vi "Dresden R2R Sputter 03.02.2018 IY24.vi"() -> ()   [LabVIEW 2009] (continued)
                                frame #1 {
                                }
                                }
                                }
                                }
                                }
                                frame #1 {
                                n30610 = stacked-sequence {
                                frame #0 {
                                n30611 = local write "Transfer_ch3_2"(TRUE ("Transfer_ch3_2")) -> ()
                                n30612 = Wait (ms)(milliseconds to wait=u32 100) -> ()  [unwired: 1 out]
                                }
                                frame #1 {
                                n30613 = while {
                                stop <- w35437 stop-if-true
                                n30614 = Wait Until Next ms Multiple(millisecond multiple=u32 300) -> ()  [unwired: 1 out]
                                n30615 = local read "Transfer_ch3_2"() -> (w35438:bool)
                                n30616 = local read "Semi"() -> (w35440:bool)
                                n30617 = Not(x=w35438) -> (.not. x?=w35439:bool)
                                n30618 = Or(x=w35439, y=w35440) -> (x .or. y?=w35437:bool)
                                }
                                }
                                }
                                }
                                frame #2 {
                                n30619 = local read "Single_Ch2_Interlock"() -> (w35441:dbl)
                                n30620 = local read "Ch2_pressure"() -> (w35445:dbl)
                                n30621 = local read "started_up_ch2"() -> (w35443:bool)
                                n30622 = In Range and Coerce(upper limit=w35441, x=w35445, lower limit=1e-08) -> (In Range?=w35446:bool)  [unwired: 1 out]
                                n30623 = And(x=w35446, y=w35443) -> (x .and. y?=w35442:bool)
                                n30624 = case shown="True" w35442 {
                                frame #0 {
                                }
                                frame #1 {
                                n30625 = local read "Semi"() -> (w35447:bool)
                                n30626 = case shown="False" w35447 {
                                frame #0 {
                                n30627 = stacked-sequence {
                                frame #0 {
                                # "WATER FLOW CONTROL OPEN"
                                n30628 = stacked-sequence {
                                frame #0 {
                                n30629 = local read "Semi"() -> (w35448:bool)
                                n30630 = case shown="False" w35448 {
                                frame #0 {
                                n30631 = while {
                                i -> [w35454]
                                stop <- w35449 stop-if-true
                                n30632 = Greater?(x=w35454, y=100) -> (0:w35453:bool)
                                n30633 = case shown="True" w35453 {
                                frame #0 {
                                }
                                frame #1 {
                                n30634 = local write "Semi"(TRUE ("Semi")) -> ()
                                n30635 = local write "Error Message"("Coating Process  \nwas cancelled.\nPlease check water \nflow connection." ("Error Message")) -> ()
                                }
                                }
                                n30636 = local read "Ch4_WFS_di"() -> (w35452:bool)
                                n30637 = case shown="True" w35452 {
                                tunnel: [TRUE FALSE] -> w35451
                                frame #0 {
                                }
                                frame #1 {
                                n30638 = local write "Ch4_WFC_do"(FALSE ("Ch1_WFC_do")) -> ()
                                n30639 = Wait Until Next ms Multiple(millisecond multiple=u32 200) -> ()  [unwired: 1 out]
                                }
                                }
                                n30640 = local read "Semi"() -> (w35450:bool)
                                n30641 = Or(x=w35451, y=w35450) -> (x .or. y?=w35449:bool)
                                }
                                }
                                frame #1 {
                                }
                                }
                                }
                                frame #1 {
                                n30642 = local read "Semi"() -> (w35462:bool)
                                n30643 = case shown="False" w35462 {
                                frame #0 {
                                n30644 = while {
                                i -> [w35468]
                                stop <- w35463 stop-if-true
                                n30645 = Greater?(x=w35468, y=100) -> (0:w35467:bool)
                                n30646 = case shown="True" w35467 {
                                frame #0 {
                                }
                                frame #1 {
                                n30647 = local write "Semi"(TRUE ("Semi")) -> ()
                                n30648 = local write "Error Message"("Coating Process  \nwas cancelled.\nPlease check water \nflow connection." ("Error Message")) -> ()
                                }
                                }
                                n30649 = local read "Ch3_WFS_di"() -> (w35466:bool)
                                n30650 = case shown="True" w35466 {
                                tunnel: [TRUE FALSE] -> w35465
                                frame #0 {
                                }
                                frame #1 {
                                n30651 = local write "Ch3_WFC_do"(FALSE ("Ch1_WFC_do")) -> ()
                                n30652 = Wait Until Next ms Multiple(millisecond multiple=u32 200) -> ()  [unwired: 1 out]
                                }
                                }
                                n30653 = local read "Semi"() -> (w35464:bool)
                                n30654 = Or(x=w35465, y=w35464) -> (x .or. y?=w35463:bool)
                                }
                                }
                                frame #1 {
                                }
                                }
                                }
                                frame #2 {
                                n30655 = local read "Semi"() -> (w35476:bool)
                                n30656 = case shown="False" w35476 {
                                frame #0 {
                                n30657 = while {
                                i -> [w35482]
                                stop <- w35477 stop-if-true
                                n30658 = Greater?(x=w35482, y=100) -> (0:w35481:bool)
                                n30659 = case shown="True" w35481 {
                                frame #0 {
                                }
                                frame #1 {
                                n30660 = local write "Semi"(TRUE ("Semi")) -> ()
                                n30661 = local write "Error Message"("Coating Process  \nwas cancelled.\nPlease check water \nflow connection." ("Error Message")) -> ()
                                }
                                }
                                n30662 = local read "Ch1_WFS_di"() -> (w35480:bool)
                                n30663 = case shown="True" w35480 {
                                tunnel: [TRUE FALSE] -> w35479
                                frame #0 {
                                }
                                frame #1 {
                                n30664 = local write "Ch1_WFC_do"(FALSE ("Ch1_WFC_do")) -> ()
                                n30665 = Wait Until Next ms Multiple(millisecond multiple=u32 200) -> ()  [unwired: 1 out]
                                }
                                }
                                n30666 = local read "Semi"() -> (w35478:bool)
                                n30667 = Or(x=w35479, y=w35478) -> (x .or. y?=w35477:bool)
                                }
                                }
                                frame #1 {
                                }
                                }
                                }
                                frame #3 {
                                n30668 = local read "Semi"() -> (w35490:bool)
                                n30669 = case shown="False" w35490 {
                                frame #0 {
                                n30670 = while {
                                i -> [w35496]
                                stop <- w35491 stop-if-true
                                n30671 = Greater?(x=w35496, y=100) -> (0:w35495:bool)
                                n30672 = case shown="True" w35495 {
                                frame #0 {
                                }
                                frame #1 {
                                n30673 = local write "Semi"(TRUE ("Semi")) -> ()
                                n30674 = local write "Error Message"("Coating Process  \nwas cancelled.\nPlease check water \nflow connection." ("Error Message")) -> ()
                                }
                                }
                                n30675 = local read "Ch2_WFS_di"() -> (w35494:bool)
                                n30676 = case shown="False" w35494 {
                                tunnel: [FALSE TRUE] -> w35493
                                frame #0 {
                                n30677 = local write "Ch2_WFC_do"(TRUE ("Ch1_WFC_do")) -> ()
                                n30678 = Wait Until Next ms Multiple(millisecond multiple=u32 200) -> ()  [unwired: 1 out]
                                }
                                frame #1 {
                                }
                                }
                                n30679 = local read "Semi"() -> (w35492:bool)
                                n30680 = Or(x=w35493, y=w35492) -> (x .or. y?=w35491:bool)
                                }
                                }
                                frame #1 {
                                }
                                }
                                }
                                frame #4 {
                                n30681 = local read "Semi"() -> (w35504:bool)
                                n30682 = case shown="False" w35504 {
                                frame #0 {
                                n30683 = local write "SDC1 2"(TRUE ("SDC1 2")) -> ()
                                n30684 = Wait (ms)(milliseconds to wait=u32 1000) -> ()  [unwired: 1 out]
                                }
                                frame #1 {
                                }
                                }
                                }
                                }
                                }
                                frame #1 {
                                # "BG-BV open"
                                n30685 = stacked-sequence {
                                frame #0 {
                                n30686 = local read "Semi"() -> (w35507:bool)
                                n30687 = case shown="False" w35507 {
                                frame #0 {
                                n30688 = while {
                                i -> [w35513]
                                stop <- w35508 stop-if-true
                                n30689 = Greater?(x=w35513, y=50) -> (0:w35512:bool)
                                n30690 = case shown="True" w35512 {
                                frame #0 {
                                }
                                frame #1 {
                                n30691 = local write "Semi"(TRUE ("Semi")) -> ()
                                n30692 = local write "Error Message"("Coating Process  \nwas cancelled.\nPlease check \nBG-BV connection." ("Error Message")) -> ()
                                }
                                }
                                n30693 = local read "Ch2_Bg_bv_di"() -> (w35511:bool)
                                n30694 = case shown="False" w35511 {
                                tunnel: [FALSE TRUE] -> w35510
                                frame #0 {
                                n30695 = local write "Ch2_Bg_bv_do"(TRUE ("Ch1_WFC_do")) -> ()
                                n30696 = Wait Until Next ms Multiple(millisecond multiple=u32 200) -> ()  [unwired: 1 out]
                                }
                                frame #1 {
                                }
                                }
                                n30697 = local read "Semi"() -> (w35509:bool)
                                n30698 = Or(x=w35510, y=w35509) -> (x .or. y?=w35508:bool)
                                }
                                }
                                frame #1 {
                                }
                                }
                                }
                                frame #1 {
                                n30699 = local read "Semi"() -> (w35521:bool)
                                n30700 = case shown="False" w35521 {
                                frame #0 {
                                n30701 = Wait (ms)(milliseconds to wait=u32 1000) -> ()  [unwired: 1 out]
                                n30702 = local write "SDC1 4"(TRUE ("SDC1 4")) -> ()
                                }
                                frame #1 {
                                }
                                }
                                }
                                }
                                }
                                frame #2 {
                                # "Baratron set zero"
                                n30703 = stacked-sequence {
                                frame #0 {
                                n30704 = local write "Pc_bv2_auto_baratron_set_zero"(TRUE ("Pc_bv2_auto_baratron_set_zero")) -> ()
                                }
                                frame #1 {
                                n30705 = while {
                                i -> [w35528]
                                stop <- w35525 stop-if-true
                                n30706 = Greater?(x=w35528, y=50 ("Baratron set zero time")) -> (0:w35527:bool)
                                n30707 = case shown="True" w35527 {
                                frame #0 {
                                }
                                frame #1 {
                                n30708 = local write "Semi"(TRUE ("Semi")) -> ()
                                n30709 = local write "Error Message"("" ("Error Message")) -> ()
                                }
                                }
                                n30710 = local read "Pressure 2"() -> (w35533:i32)
                                n30711 = Less?(x=w35533, y=0.1 ("Pressure Check for baratron set zero")) -> (x < y?=w35531:bool)
                                n30712 = case shown="False" w35531 {
                                tunnel: [FALSE TRUE] -> w35530
                                frame #0 {
                                n30713 = Wait Until Next ms Multiple(millisecond multiple=u32 200) -> ()  [unwired: 1 out]
                                }
                                frame #1 {
                                }
                                }
                                n30714 = local read "Semi"() -> (w35529:bool)
                                n30715 = Or(x=w35530, y=w35529) -> (x .or. y?=w35525:bool)
                                }
                                }
                                frame #2 {
                                n30716 = local read "Semi"() -> (w35539:bool)
                                n30717 = case shown="False" w35539 {
                                frame #0 {
                                n30718 = local write "SDC1 2b"(TRUE ("SDC1 2b")) -> ()
                                n30719 = Wait (ms)(milliseconds to wait=u32 1000) -> ()  [unwired: 1 out]
                                }
                                frame #1 {
                                }
                                }
                                }
                                }
                                }
                                frame #3 {
                                # "CC CLOSE"
                                n30720 = stacked-sequence {
                                frame #0 {
                                n30721 = local read "Semi"() -> (w35542:bool)
                                n30722 = case shown="False" w35542 {
                                frame #0 {
                                n30723 = while {
                                i -> [w35548]
                                stop <- w35543 stop-if-true
                                n30724 = Greater?(x=w35548, y=50) -> (0:w35547:bool)
                                n30725 = case shown="True" w35547 {
                                frame #0 {
                                }
                                frame #1 {
                                n30726 = local write "Semi"(TRUE ("Semi")) -> ()
                                n30727 = local write "Error Message"("Coating Process  \nwas cancelled.\nPlease check \nBG-BV connection." ("Error Message")) -> ()
                                }
                                }
                                n30728 = local read "Ch2_Cc_on_off_di"() -> (w35546:bool)
                                n30729 = case shown="True" w35546 {
                                tunnel: [TRUE FALSE] -> w35545
                                frame #0 {
                                }
                                frame #1 {
                                n30730 = local write "Ch2_Cc_on_off_do"(FALSE ("Ch1_WFC_do")) -> ()
                                n30731 = Wait Until Next ms Multiple(millisecond multiple=u32 200) -> ()  [unwired: 1 out]
                                }
                                }
                                n30732 = local read "Semi"() -> (w35544:bool)
                                n30733 = Or(x=w35545, y=w35544) -> (x .or. y?=w35543:bool)
                                }
                                }
                                frame #1 {
                                }
                                }
                                }
                                frame #1 {
                                n30734 = local read "Semi"() -> (w35556:bool)
                                n30735 = case shown="False" w35556 {
                                frame #0 {
                                n30736 = local write "SDC1 3"(TRUE ("SDC1 3")) -> ()
                                n30737 = Wait (ms)(milliseconds to wait=u32 1000) -> ()  [unwired: 1 out]
                                }
                                frame #1 {
                                }
                                }
                                }
                                }
                                }
                                frame #4 {
                                # "PC-BV CLOSE"
                                n30738 = stacked-sequence {
                                frame #0 {
                                n30739 = local read "Semi"() -> (w35559:bool)
                                n30740 = case shown="False" w35559 {
                                frame #0 {
                                n30741 = stacked-sequence {
                                frame #0 {
                                n30742 = local read "Semi"() -> (w35560:bool)
                                n30743 = case shown="False" w35560 {
                                frame #0 {
                                n30744 = local write "Pc_bv2_auto_close"(TRUE ("Tp1_auto_start")) -> ()
                                }
                                frame #1 {
                                }
                                }
                                }
                                frame #1 {
                                n30745 = local read "Semi"() -> (w35562:bool)
                                n30746 = case shown="False" w35562 {
                                frame #0 {
                                n30747 = Wait (ms)(milliseconds to wait=u32 1000) -> ()  [unwired: 1 out]
                                }
                                frame #1 {
                                }
                                }
                                }
                                frame #2 {
                                n30748 = local read "Semi"() -> (w35564:bool)
                                n30749 = case shown="False" w35564 {
                                frame #0 {
                                n30750 = while {
                                i -> [w35570]
                                stop <- w35566 stop-if-true
                                n30751 = local read "Pc_bv_closed_ch2"() -> (w35568:bool)
                                n30752 = Greater?(x=w35570, y=120) -> (0:w35569:bool)
                                n30753 = local read "Semi"() -> (w35567:bool)
                                n30754 = Compound Arithmetic op=OR(w35567, w35568, w35569) -> (w35566:bool)
                                n30755 = Wait (ms)(milliseconds to wait=u32 500) -> ()  [unwired: 1 out]
                                }
                                }
                                frame #1 {
                                }
                                }
                                }
                                frame #3 {
                                n30756 = local read "Semi"() -> (w35572:bool)
                                n30757 = case shown="False" w35572 {
                                frame #0 {
                                n30758 = local read "Pc_bv_closed_ch2"() -> (w35573:bool)
                                n30759 = case shown="False" w35573 {
                                frame #0 {
                                n30760 = local write "Pc_bv2_auto_close"(TRUE ("Pc_bv1_auto_open")) -> ()
                                }
                                frame #1 {
                                }
                                }
                                }
                                frame #1 {
                                }
                                }
                                }
                                frame #4 {
                                n30761 = local read "Semi"() -> (w35575:bool)
                                n30762 = case shown="False" w35575 {
                                frame #0 {
                                n30763 = local read "Pc_bv_closed_ch2"() -> (w35576:bool)
                                n30764 = case shown="False" w35576 {
                                frame #0 {
                                n30765 = Wait (ms)(milliseconds to wait=u32 1000) -> ()  [unwired: 1 out]
                                }
                                frame #1 {
                                }
                                }
                                }
                                frame #1 {
                                }
                                }
                                }
                                frame #5 {
                                n30766 = local read "Semi"() -> (w35578:bool)
                                n30767 = case shown="False" w35578 {
                                frame #0 {
                                n30768 = while {
                                i -> [w35584]
                                stop <- w35580 stop-if-true
                                n30769 = local read "Pc_bv_closed_ch2"() -> (w35582:bool)
                                n30770 = Greater?(x=w35584, y=120) -> (0:w35583:bool)
                                n30771 = local read "Semi"() -> (w35581:bool)
                                n30772 = Compound Arithmetic op=OR(w35581, w35582, w35583) -> (w35580:bool)
                                n30773 = Wait (ms)(milliseconds to wait=u32 500) -> ()  [unwired: 1 out]
                                }
                                }
                                frame #1 {
                                }
                                }
                                }
                                frame #6 {
                                n30774 = local read "Semi"() -> (w35586:bool)
                                n30775 = case shown="False" w35586 {
                                frame #0 {
                                n30776 = local read "Pc_bv_closed_ch2"() -> (w35587:bool)
                                n30777 = case shown="False" w35587 {
                                frame #0 {
                                n30778 = local write "Error Message"("Start up process  cancelled\nbecause  PC-BV not closed.\nPlease check PC-BV1 connections." ("Error Message")) -> ()
                                n30779 = Wait (ms)(milliseconds to wait=u32 1000) -> ()  [unwired: 1 out]
                                }
                                frame #1 {
                                }
                                }
                                }
                                frame #1 {
                                }
                                }
                                }
                                }
                                }
                                frame #1 {
                                }
                                }
                                }
                                frame #1 {
                                n30780 = local read "Semi"() -> (w35590:bool)
                                n30781 = case shown="False" w35590 {
                                frame #0 {
                                n30782 = local write "SDC1 5"(TRUE ("SDC1 5")) -> ()
                                n30783 = Wait (ms)(milliseconds to wait=u32 1000) -> ()  [unwired: 1 out]
                                }
                                frame #1 {
                                }
                                }
                                }
                                }
                                }
                                frame #5 {
                                # "SOV-AR OPEN"
                                n30784 = stacked-sequence {
                                frame #0 {
                                n30785 = local read "Semi"() -> (w35593:bool)
                                n30786 = case shown="False" w35593 {
                                frame #0 {
                                n30787 = while {
                                i -> [w35599]
                                stop <- w35594 stop-if-true
                                n30788 = Greater?(x=w35599, y=50) -> (0:w35598:bool)
                                n30789 = case shown="True" w35598 {
                                frame #0 {
                                }
                                frame #1 {
                                n30790 = local write "Semi"(TRUE ("Semi")) -> ()
                                n30791 = local write "Error Message"("Coating Process  \nwas cancelled.\nPlease check \nSOV-Ar connection." ("Error Message")) -> ()
                                }
                                }
                                n30792 = local read "Ch2_Sov_Ar_di"() -> (w35597:bool)
                                n30793 = case shown="False" w35597 {
                                tunnel: [FALSE TRUE] -> w35596
                                frame #0 {
                                n30794 = local write "Ch2_Sov_Ar_do"(TRUE ("Ch1_WFC_do")) -> ()
                                n30795 = Wait Until Next ms Multiple(millisecond multiple=u32 200) -> ()  [unwired: 1 out]
                                }
                                frame #1 {
                                }
                                }
                                n30796 = local read "Semi"() -> (w35595:bool)
                                n30797 = Or(x=w35596, y=w35595) -> (x .or. y?=w35594:bool)
                                }
                                }
                                frame #1 {
                                }
                                }
                                }
                                frame #1 {
                                n30798 = local read "Semi"() -> (w35607:bool)
                                n30799 = case shown="False" w35607 {
                                frame #0 {
                                n30800 = while {
                                i -> [w35612]
                                stop <- w35610 stop-if-true
                                n30801 = Greater?(x=w35612, y=5) -> (0:w35608:bool)
                                n30802 = Wait Until Next ms Multiple(millisecond multiple=u32 1000) -> ()  [unwired: 1 out]
                                n30803 = local read "Semi"() -> (w35611:bool)
                                n30804 = Or(x=w35608, y=w35611) -> (x .or. y?=w35610:bool)
                                }
                                }
                                frame #1 {
                                }
                                }
                                }
                                frame #2 {
                                n30805 = local read "Semi"() -> (w35614:bool)
                                n30806 = case shown="False" w35614 {
                                frame #0 {
                                n30807 = local write "SDC1 6"(TRUE ("SDC1 6")) -> ()
                                n30808 = Wait (ms)(milliseconds to wait=u32 1000) -> ()  [unwired: 1 out]
                                }
                                frame #1 {
                                }
                                }
                                }
                                }
                                }
                                frame #6 {
                                # "CHECK CHAMBER PRESSURE"
                                n30809 = stacked-sequence {
                                frame #0 {
                                n30810 = local read "Semi"() -> (w35617:bool)
                                n30811 = case shown="False" w35617 {
                                frame #0 {
                                n30812 = while {
                                i -> [w35625]
                                stop <- w35619 stop-if-true
                                n30813 = Greater?(x=w35625, y=300) -> (0:w35624:bool)
                                n30814 = case shown="True" w35624 {
                                frame #0 {
                                }
                                frame #1 {
                                n30815 = local write "Semi"(TRUE ("Semi")) -> ()
                                n30816 = local write "Error Message"("Coating Process cancelled.\nPlease check chamber \nconnections." ("Error Message")) -> ()
                                }
                                }
                                n30817 = local read "Ch_pg_press_ch2_gui 2"() -> (w35618:dbl)
                                n30818 = Greater Or Equal?(x=w35618, y=0.9 ("CHAMBER PRESSURE 4")) -> (x >= y?=w35622:bool)
                                n30819 = case shown="True" w35622 {
                                tunnel: [TRUE FALSE] -> w35621
                                frame #0 {
                                }
                                frame #1 {
                                n30820 = Wait Until Next ms Multiple(millisecond multiple=u32 200) -> ()  [unwired: 1 out]
                                }
                                }
                                n30821 = local read "Semi"() -> (w35620:bool)
                                n30822 = Or(x=w35621, y=w35620) -> (x .or. y?=w35619:bool)
                                }
                                }
                                frame #1 {
                                }
                                }
                                }
                                frame #1 {
                                n30823 = local read "Semi"() -> (w35632:bool)
                                n30824 = case shown="False" w35632 {
                                frame #0 {
                                n30825 = Wait (ms)(milliseconds to wait=u32 1000) -> ()  [unwired: 1 out]
                                n30826 = local write "SDC1 8"(TRUE ("SDC1 8")) -> ()
                                }
                                frame #1 {
                                }
                                }
                                }
                                }
                                }
                                frame #7 {
                                # "PC-BV OPEN"
                                n30827 = stacked-sequence {
                                frame #0 {
                                n30828 = local read "Semi"() -> (w35635:bool)
                                n30829 = case shown="False" w35635 {
                                frame #0 {
                                n30830 = stacked-sequence {
                                frame #0 {
                                n30831 = local read "Semi"() -> (w35636:bool)
                                n30832 = case shown="False" w35636 {
                                frame #0 {
                                n30833 = local write "Pc_bv2_auto_open"(TRUE ("Tp1_auto_start")) -> ()
                                }
                                frame #1 {
                                }
                                }
                                }
                                frame #1 {
                                n30834 = local read "Semi"() -> (w35638:bool)
                                n30835 = case shown="False" w35638 {
                                frame #0 {
                                n30836 = Wait (ms)(milliseconds to wait=u32 1000) -> ()  [unwired: 1 out]
                                }
                                frame #1 {
                                }
                                }
                                }
                                frame #2 {
                                n30837 = local read "Semi"() -> (w35640:bool)
                                n30838 = case shown="False" w35640 {
                                frame #0 {
                                n30839 = while {
                                i -> [w35646]
                                stop <- w35642 stop-if-true
                                n30840 = local read "Pc_bv_opened_ch2"() -> (w35644:bool)
                                n30841 = Greater?(x=w35646, y=120) -> (0:w35645:bool)
                                n30842 = local read "Semi"() -> (w35643:bool)
                                n30843 = Compound Arithmetic op=OR(w35643, w35644, w35645) -> (w35642:bool)
                                n30844 = Wait (ms)(milliseconds to wait=u32 500) -> ()  [unwired: 1 out]
                                }
                                }
                                frame #1 {
                                }
                                }
                                }
                                frame #3 {
                                n30845 = local read "Semi"() -> (w35648:bool)
                                n30846 = case shown="False" w35648 {
                                frame #0 {
                                n30847 = local read "Pc_bv_opened_ch2"() -> (w35649:bool)
                                n30848 = case shown="False" w35649 {
                                frame #0 {
                                n30849 = local write "Pc_bv2_auto_open"(TRUE ("Pc_bv1_auto_open")) -> ()
                                }
                                frame #1 {
                                }
                                }
                                }
                                frame #1 {
                                }
                                }
                                }
                                frame #4 {
                                n30850 = local read "Semi"() -> (w35651:bool)
                                n30851 = case shown="False" w35651 {
                                frame #0 {
                                n30852 = local read "Pc_bv_opened_ch2"() -> (w35652:bool)
                                n30853 = case shown="False" w35652 {
                                frame #0 {
                                n30854 = Wait (ms)(milliseconds to wait=u32 1000) -> ()  [unwired: 1 out]
                                }
                                frame #1 {
                                }
                                }
                                }
                                frame #1 {
                                }
                                }
                                }
                                frame #5 {
                                n30855 = local read "Semi"() -> (w35654:bool)
                                n30856 = case shown="False" w35654 {
                                frame #0 {
                                n30857 = while {
                                i -> [w35660]
                                stop <- w35656 stop-if-true
                                n30858 = local read "Pc_bv_opened_ch2"() -> (w35658:bool)
                                n30859 = Greater?(x=w35660, y=120) -> (0:w35659:bool)
                                n30860 = local read "Semi"() -> (w35657:bool)
                                n30861 = Compound Arithmetic op=OR(w35657, w35658, w35659) -> (w35656:bool)
                                n30862 = Wait (ms)(milliseconds to wait=u32 500) -> ()  [unwired: 1 out]
                                }
                                }
                                frame #1 {
                                }
                                }
                                }
                                frame #6 {
                                n30863 = local read "Semi"() -> (w35662:bool)
                                n30864 = case shown="False" w35662 {
                                frame #0 {
                                n30865 = local read "Pc_bv_opened_ch2"() -> (w35663:bool)
                                n30866 = case shown="False" w35663 {
                                frame #0 {
                                n30867 = local write "Error Message"("Start up process  cancelled\nbecause  PC-BV not opened.\nPlease check PC-BV1 connections." ("Error Message")) -> ()
                                n30868 = Wait (ms)(milliseconds to wait=u32 1000) -> ()  [unwired: 1 out]
                                }
                                frame #1 {
                                }
                                }
                                }
                                frame #1 {
                                }
                                }
                                }
                                }
                                }
                                frame #1 {
                                }
                                }
                                }
                                frame #1 {
                                n30869 = local read "Semi"() -> (w35666:bool)
                                n30870 = case shown="False" w35666 {
                                frame #0 {
                                n30871 = Wait (ms)(milliseconds to wait=u32 1000) -> ()  [unwired: 1 out]
                                n30872 = local write "SDC1 7"(TRUE ("SDC1 7")) -> ()
                                }
                                frame #1 {
                                }
                                }
                                }
                                }
                                }
                                frame #8 {
                                # "CC OPEN"
                                n30873 = stacked-sequence {
                                frame #0 {
                                n30874 = local read "Semi"() -> (w35669:bool)
                                n30875 = case shown="False" w35669 {
                                frame #0 {
                                n30876 = while {
                                i -> [w35675]
                                stop <- w35670 stop-if-true
                                n30877 = Greater?(x=w35675, y=50) -> (0:w35674:bool)
                                n30878 = case shown="True" w35674 {
                                frame #0 {
                                }
                                frame #1 {
                                n30879 = local write "Semi"(TRUE ("Semi")) -> ()
                                n30880 = local write "Error Message"("Coating Process  \nwas cancelled.\nPlease check \nBG-BV connection." ("Error Message")) -> ()
                                }
                                }
                                n30881 = local read "Ch2_Cc_on_off_di"() -> (w35673:bool)
                                n30882 = case shown="True" w35673 {
                                tunnel: [FALSE TRUE] -> w35672
                                frame #0 {
                                n30883 = local write "Ch2_Cc_on_off_do"(TRUE ("Ch1_WFC_do")) -> ()
                                n30884 = Wait Until Next ms Multiple(millisecond multiple=u32 200) -> ()  [unwired: 1 out]
                                }
                                frame #1 {
                                }
                                }
                                n30885 = local read "Semi"() -> (w35671:bool)
                                n30886 = Or(x=w35672, y=w35671) -> (x .or. y?=w35670:bool)
                                }
                                }
                                frame #1 {
                                }
                                }
                                }
                                frame #1 {
                                n30887 = local read "Semi"() -> (w35683:bool)
                                n30888 = case shown="False" w35683 {
                                frame #0 {
                                n30889 = while {
                                i -> [w35688]
                                stop <- w35686 stop-if-true
                                n30890 = Greater?(x=w35688, y=30) -> (0:w35684:bool)
                                n30891 = Wait Until Next ms Multiple(millisecond multiple=u32 1000) -> ()  [unwired: 1 out]
                                n30892 = local read "Semi"() -> (w35687:bool)
                                n30893 = Or(x=w35684, y=w35687) -> (x .or. y?=w35686:bool)
                                }
                                }
                                frame #1 {
                                }
                                }
                                }
                                frame #2 {
                                n30894 = local read "Semi"() -> (w35690:bool)
                                n30895 = case shown="False" w35690 {
                                frame #0 {
                                n30896 = Wait (ms)(milliseconds to wait=u32 1000) -> ()  [unwired: 1 out]
                                n30897 = local write "SDC1 7b"(TRUE ("SDC1 3")) -> ()
                                }
                                frame #1 {
                                }
                                }
                                }
                                }
                                }
                                frame #9 {
                                # "CHECK CHAMBER PRESSURE"
                                n30898 = stacked-sequence {
                                frame #0 {
                                n30899 = local read "Semi"() -> (w35693:bool)
                                n30900 = case shown="False" w35693 {
                                frame #0 {
                                n30901 = while {
                                i -> [w35701]
                                stop <- w35695 stop-if-true
                                n30902 = Greater?(x=w35701, y=300) -> (0:w35700:bool)